vi "singleChannelGraphs_1.vi"(8 "Locations-IR 2":dbl[][](array[numeric])=[[0.0, 0.0, 0.0, 0.0, 0.0, 0.0, 0.0, 0.0, 0.0, 0.0, 0.0], [0.0, 0.0, 0.0, 0.0, 0.0, 0.0, 0.0, 0.0, 0.0, 0.0, 0.0], [0.0, 0.0, 0.0, 0.0, 0.0, 0.0, 0.0, 0.0, 0.0, 0.0, 0.0], [0.0, 0.0, 0.0, 0.0, 0.0, 0.0, 0.0, 0.0, 0.0, 0.0, 0.0], [1003.5977793333972, 1010.2987872733909, 1047.7043573372093, 1054.0581575907959, 1060.2441183129574, 1066.4237494286472, 1072.6076798246322, 1078.8502256474524, 1119.8606859005151, 1131.4795052552802, 1142.8109565689153], [0.0, 0.0, 0.0, 0.0, 0.0, 0.0, 0.0, 0.0, 0.0, 0.0, 0.0], [8947.909400008684, 0.0, 0.0, 0.0, 0.0, 0.0, 0.0, 0.0, 0.0, 0.0, 0.0], [0.0, 0.0, 0.0, 0.0, 0.0, 0.0, 0.0, 0.0, 0.0, 0.0, 0.0], [0.0, 0.0, 0.0, 0.0, 0.0, 0.0, 0.0, 0.0, 0.0, 0.0, 0.0], [0.0, 0.0, 0.0, 0.0, 0.0, 0.0, 0.0, 0.0, 0.0, 0.0, 0.0], [0.0, 0.0, 0.0, 0.0, 0.0, 0.0, 0.0, 0.0, 0.0, 0.0, 0.0], [0.0, 0.0, 0.0, 0.0, 0.0, 0.0, 0.0, 0.0, 0.0, 0.0, 0.0], [0.0, 0.0, 0.0, 0.0, 0.0, 0.0, 0.0, 0.0, 0.0, 0.0, 0.0], [0.0, 0.0, 0.0, 0.0, 0.0, 0.0, 0.0, 0.0, 0.0, 0.0, 0.0]], 9 "Locations-IR 1":dbl[][](array[numeric])=[[0.0, 0.0, 0.0, 0.0, 0.0, 0.0, 0.0, 0.0, 0.0, 0.0, 0.0, 0.0, 0.0, 0.0, 0.0, 0.0, 0.0, 0.0, 0.0, 0.0, 0.0, 0.0, 0.0, 0.0], [0.0, 0.0, 0.0, 0.0, 0.0, 0.0, 0.0, 0.0, 0.0, 0.0, 0.0, 0.0, 0.0, 0.0, 0.0, 0.0, 0.0, 0.0, 0.0, 0.0, 0.0, 0.0, 0.0, 0.0], [0.0, 0.0, 0.0, 0.0, 0.0, 0.0, 0.0, 0.0, 0.0, 0.0, 0.0, 0.0, 0.0, 0.0, 0.0, 0.0, 0.0, 0.0, 0.0, 0.0, 0.0, 0.0, 0.0, 0.0], [0.0, 0.0, 0.0, 0.0, 0.0, 0.0, 0.0, 0.0, 0.0, 0.0, 0.0, 0.0, 0.0, 0.0, 0.0, 0.0, 0.0, 0.0, 0.0, 0.0, 0.0, 0.0, 0.0, 0.0], [0.0, 0.0, 0.0, 0.0, 0.0, 0.0, 0.0, 0.0, 0.0, 0.0, 0.0, 0.0, 0.0, 0.0, 0.0, 0.0, 0.0, 0.0, 0.0, 0.0, 0.0, 0.0, 0.0, 0.0], [1949.3968989382124, 8950.779704911463, 0.0, 0.0, 0.0, 0.0, 0.0, 0.0, 0.0, 0.0, 0.0, 0.0, 0.0, 0.0, 0.0, 0.0, 0.0, 0.0, 0.0, 0.0, 0.0, 0.0, 0.0, 0.0], [1922.6824130689417, 1927.4536577782014, 8945.1544536163, 0.0, 0.0, 0.0, 0.0, 0.0, 0.0, 0.0, 0.0, 0.0, 0.0, 0.0, 0.0, 0.0, 0.0, 0.0, 0.0, 0.0, 0.0, 0.0, 0.0, 0.0], [8944.05693493819, 0.0, 0.0, 0.0, 0.0, 0.0, 0.0, 0.0, 0.0, 0.0, 0.0, 0.0, 0.0, 0.0, 0.0, 0.0, 0.0, 0.0, 0.0, 0.0, 0.0, 0.0, 0.0, 0.0], [1828.0609508803298, 1840.7040446097299, 1846.0822777647768, 1851.546050134507, 1859.188023533712, 1880.890963654859, 8946.459150564613, 0.0, 0.0, 0.0, 0.0, 0.0, 0.0, 0.0, 0.0, 0.0, 0.0, 0.0, 0.0, 0.0, 0.0, 0.0, 0.0, 0.0], [1003.8836135739322, 1034.6023970013964, 1053.8529427226035, 1059.3332515391548, 1066.1957876120568, 1101.2443464523667, 1107.1271826334205, 1113.3003458195556, 1124.7988705144635, 1158.4306678463795, 1163.8291284517709, 1174.9323436186403, 1222.5151135054907, 1227.7098546004795, 1278.1537733001408, 1789.4645001942506, 1803.3995277539998, 1813.0755151476708, 1815.1158947507906, 1827.5667796787511, 1840.7614524568564, 7629.760547014096, 8952.76455905497, 9371.69731664426], [1786.270481148661, 1790.662343187161, 1799.7774170223831, 0.0, 0.0, 0.0, 0.0, 0.0, 0.0, 0.0, 0.0, 0.0, 0.0, 0.0, 0.0, 0.0, 0.0, 0.0, 0.0, 0.0, 0.0, 0.0, 0.0, 0.0], [1758.269290749024, 1768.7972022285298, 1773.1698271444452, 1779.905620445401, 1785.2748566498417, 1797.4164166157257, 0.0, 0.0, 0.0, 0.0, 0.0, 0.0, 0.0, 0.0, 0.0, 0.0, 0.0, 0.0, 0.0, 0.0, 0.0, 0.0, 0.0, 0.0], [1731.9130549197157, 1741.9528957065543, 1746.8638380092243, 1756.4292982249558, 1769.4936601847248, 1775.4511666930466, 1785.5242437749614, 0.0, 0.0, 0.0, 0.0, 0.0, 0.0, 0.0, 0.0, 0.0, 0.0, 0.0, 0.0, 0.0, 0.0, 0.0, 0.0, 0.0], [1670.107666290024, 1721.118225421893, 1731.7339852624614, 1741.1929011419254, 1747.322588791405, 1755.3693388267866, 1763.3171095427958, 1768.6483249049165, 0.0, 0.0, 0.0, 0.0, 0.0, 0.0, 0.0, 0.0, 0.0, 0.0, 0.0, 0.0, 0.0, 0.0, 0.0, 0.0]], 10 "micro 1":dbl[][](array[numeric])=array14x10000[140000 elements], 11 "micro 2":dbl[][](array[numeric])=array14x10000[140000 elements]) -> ()   [LabVIEW 2014]
panel:
  in  "Numerisch":i32=30
  in  "Registerkarte":enum32{"micro 2", "micro 1"}(tab)=enum."micro 1"
  out "Gap_L11":dbl[][](graph)
  out "Gap_L10":dbl[][](graph)
  out "Gap_L9":dbl[][](graph)
  out "Gap_L8":dbl[][](graph)
  out "Gap_L7":dbl[][](graph)
  out "Gap_L6":dbl[][](graph)
  out "Gap_L5":dbl[][](graph)
  out "Gap_L4":dbl[][](graph)
  out "Gap_L3":dbl[][](graph)
  out "Gap_L1":dbl[][](graph)
  out "Gap_L2":dbl[][](graph)
  out "Gap_L12":dbl[][](graph)
  out "Gap_L13":dbl[][](graph)
  out "Gap_L14":dbl[][](graph)
  out "Gap_R11":dbl[][](graph)
  out "Gap_R10":dbl[][](graph)
  out "Gap_R9":dbl[][](graph)
  out "Gap_R8":dbl[][](graph)
  out "Gap_R6":dbl[][](graph)
  out "Gap_R5":dbl[][](graph)
  out "Gap_R4":dbl[][](graph)
  out "Speaker R3":dbl[][](graph)
  out "Gap_R7":dbl[][](graph)
  out "Speaker R1":dbl[](graph)
  out "Speaker R2":dbl[](graph)
  out "Speaker R14":dbl[](graph)
  out "Gap_R11 2":dbl[][](graph)
  out "Gap_R13":dbl[][](graph)
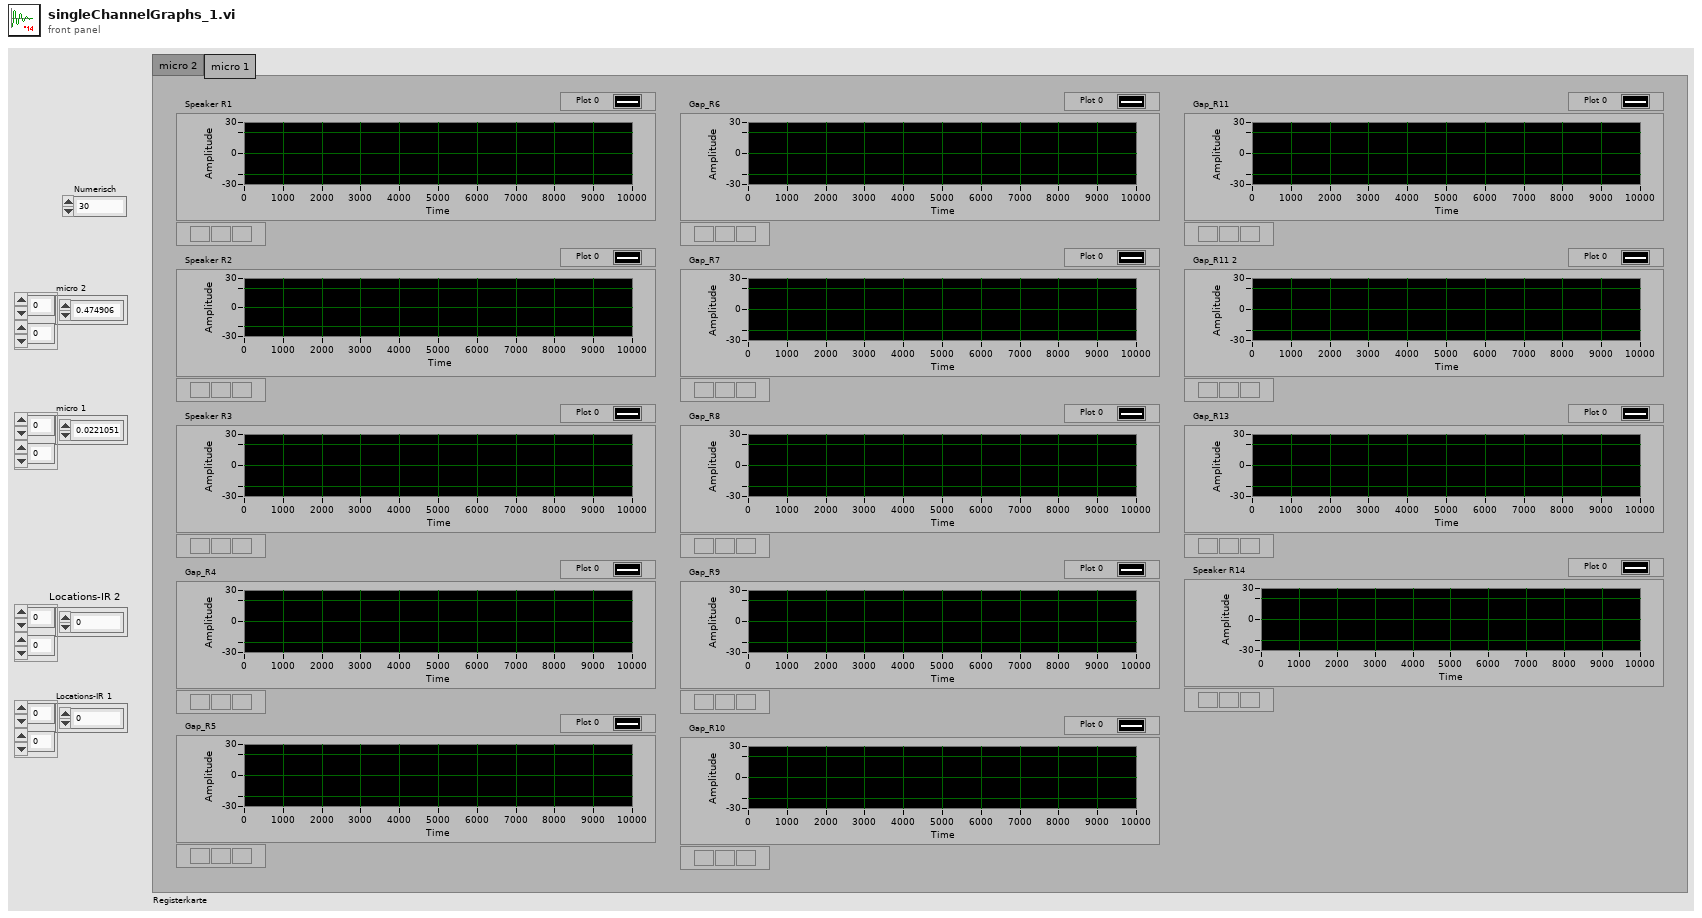
[diagram p1: front panel]
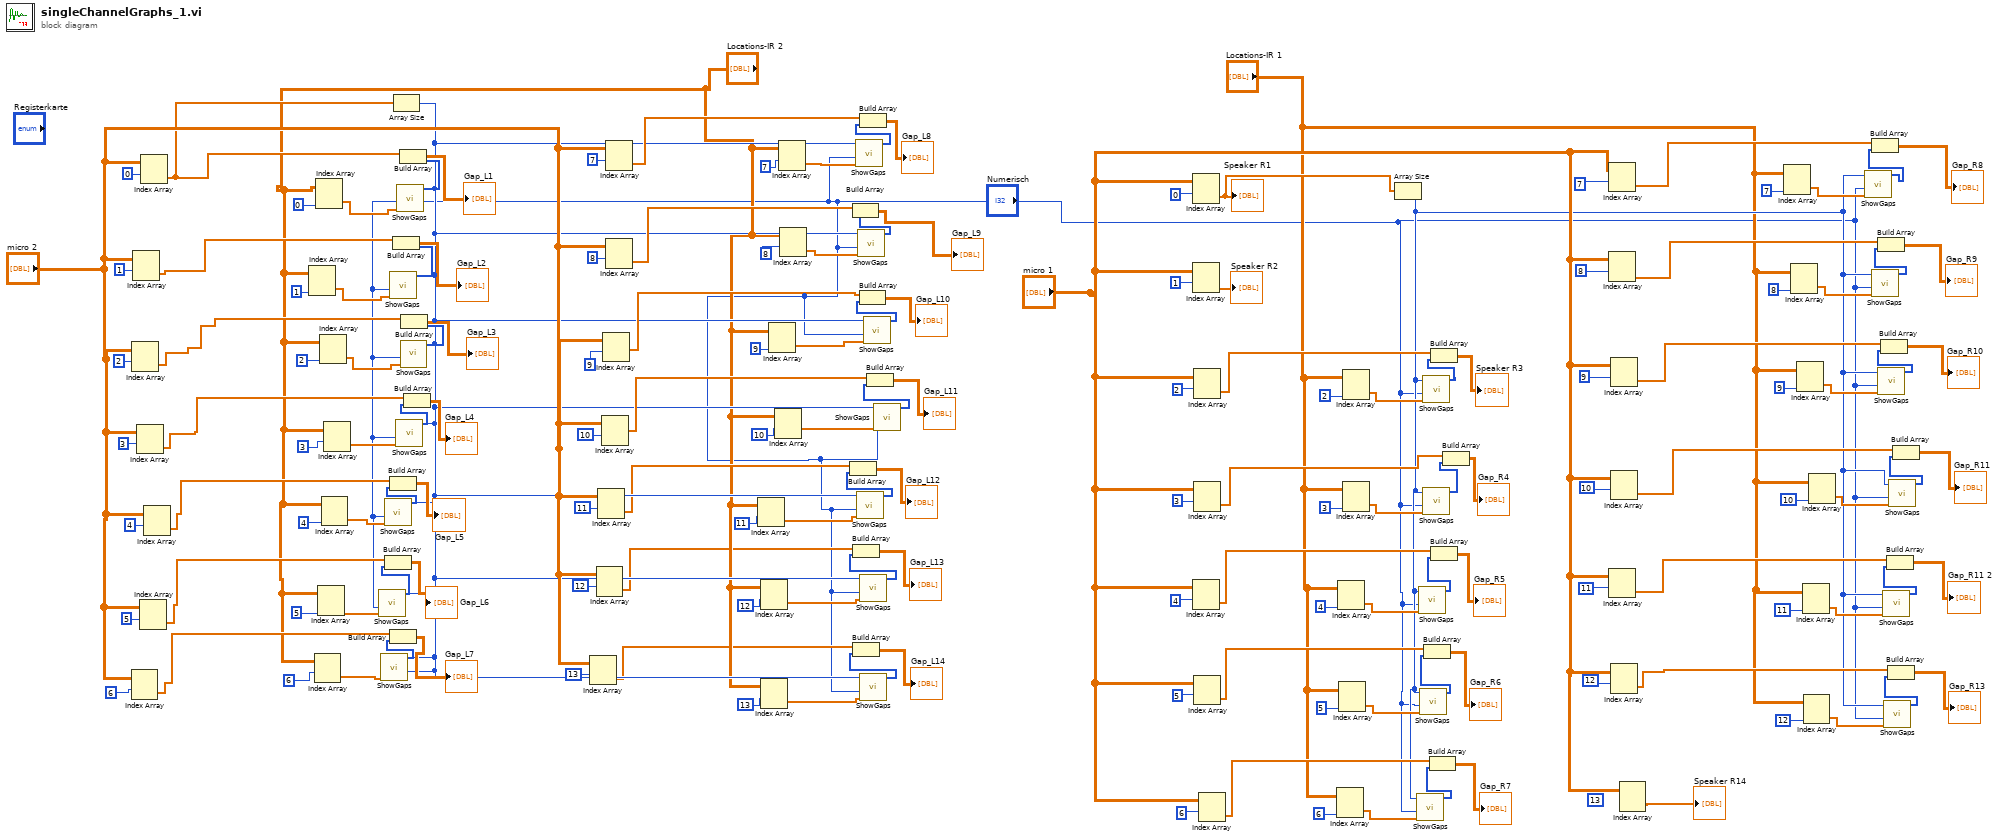
[diagram p0: block diagram]
diagram:
  (unwired) 13
  n1 = Index Array(array="micro 2", index (row)=6) -> (element=w82:dbl[])  [unwired: 1 in]
  n2 = Index Array(array="micro 2", index (row)=2) -> (element=w94:dbl[])  [unwired: 1 in]
  n3 = Index Array(array="micro 2", index (row)=1) -> (element=w20:dbl[])  [unwired: 1 in]
  n4 = Index Array(array="micro 2", index (row)=3) -> (element=w91:dbl[])  [unwired: 1 in]
  n5 = Index Array(array="micro 2", index (row)=5) -> (element=w85:dbl[])  [unwired: 1 in]
  n6 = Index Array(array="micro 2", index (row)=0) -> (element=w21:dbl[])  [unwired: 1 in]
  n7 = Index Array(array="micro 2", index (row)=4) -> (element=w88:dbl[])  [unwired: 1 in]
  n8 = Index Array(array="Locations-IR 2", index (row)=1 ("Index (Spalte)")) -> (element=w24:dbl[])  [unwired: 1 in]
  n9 = Index Array(array="Locations-IR 2", index (row)=6 ("Index (Spalte)")) -> (element=w118:dbl[])  [unwired: 1 in]
  n10 = Index Array(array="Locations-IR 2", index (row)=0 ("Index (Spalte)")) -> (element=w27:dbl[])  [unwired: 1 in]
  n11 = Index Array(array="Locations-IR 2", index (row)=5 ("Index (Spalte)")) -> (element=w119:dbl[])  [unwired: 1 in]
  n12 = Index Array(array="Locations-IR 2", index (row)=2 ("Index (Spalte)")) -> (element=w122:dbl[])  [unwired: 1 in]
  n13 = Index Array(array="Locations-IR 2", index (row)=4 ("Index (Spalte)")) -> (element=w120:dbl[])  [unwired: 1 in]
  n14 = Index Array(array="Locations-IR 2", index (row)=3 ("Index (Spalte)")) -> (element=w121:dbl[])  [unwired: 1 in]
  n15 = Array Size(array=w21) -> (size(s)=w9:i32)
  n16 = call "ShowGaps.vi"("peaklocations"=w119, "Numerisch"="Numerisch", "length of IR"=w9) -> ("ShowGap"=w84:i32[])  [unwired: 8 in]
  n17 = call "ShowGaps.vi"("peaklocations"=w118, "Numerisch"=w9, "length of IR"=w9) -> ("ShowGap"=w81:i32[])  [unwired: 8 in]
  n18 = call "ShowGaps.vi"("peaklocations"=w120, "Numerisch"="Numerisch", "length of IR"=w9) -> ("ShowGap"=w87:i32[])  [unwired: 8 in]
  n19 = Build Array(w85, w84) -> (→"Gap_L6":dbl[][])
  n20 = call "ShowGaps.vi"("peaklocations"=w24, "Numerisch"="Numerisch", "length of IR"=w9) -> ("ShowGap"=w23:i32[])  [unwired: 8 in]
  n21 = Build Array(w88, w87) -> (→"Gap_L5":dbl[][])
  n22 = Build Array(w82, w81) -> (→"Gap_L7":dbl[][])
  n23 = Build Array(w20, w23) -> (→"Gap_L2":dbl[][])
  n24 = call "ShowGaps.vi"("peaklocations"=w121, "Numerisch"="Numerisch", "length of IR"=w9) -> ("ShowGap"=w90:i32[])  [unwired: 8 in]
  n25 = call "ShowGaps.vi"("peaklocations"=w27, "length of IR"=w9) -> ("ShowGap"=w26:i32[])  [unwired: 9 in]
  n26 = Build Array(w21, w26) -> (→"Gap_L1":dbl[][])
  n27 = call "ShowGaps.vi"("peaklocations"=w122, "Numerisch"="Numerisch", "length of IR"=w9) -> ("ShowGap"=w93:i32[])  [unwired: 8 in]
  n28 = Build Array(w94, w93) -> (→"Gap_L3":dbl[][])
  n29 = Build Array(w91, w90) -> (→"Gap_L4":dbl[][])
  n30 = Index Array(array="micro 2", index (row)=13) -> (element=w6:dbl[])  [unwired: 1 in]
  n31 = Index Array(array="micro 2", index (row)=12) -> (element=w5:dbl[])  [unwired: 1 in]
  n32 = Index Array(array="micro 2", index (row)=11) -> (element=w8:dbl[])  [unwired: 1 in]
  n33 = Index Array(array="micro 2", index (row)=10) -> (element=w70:dbl[])  [unwired: 1 in]
  n34 = Index Array(array="micro 2", index (row)=9) -> (element=w73:dbl[])  [unwired: 1 in]
  n35 = Index Array(array="micro 2", index (row)=7) -> (element=w79:dbl[])  [unwired: 1 in]
  n36 = Index Array(array="micro 2", index (row)=8) -> (element=w76:dbl[])  [unwired: 1 in]
  n37 = Index Array(array="Locations-IR 2", index (row)=11 ("Index (Spalte)")) -> (element=w3:dbl[])  [unwired: 1 in]
  n38 = Index Array(array="Locations-IR 2", index (row)=12 ("Index (Spalte)")) -> (element=w4:dbl[])  [unwired: 1 in]
  n39 = Index Array(array="Locations-IR 2", index (row)=13 ("Index (Spalte)")) -> (element=w2:dbl[])  [unwired: 1 in]
  n40 = Index Array(array="Locations-IR 2", index (row)=9 ("Index (Spalte)")) -> (element=w116:dbl[])  [unwired: 1 in]
  n41 = Index Array(array="Locations-IR 2", index (row)=10 ("Index (Spalte)")) -> (element=w117:dbl[])  [unwired: 1 in]
  n42 = Index Array(array="Locations-IR 2", index (row)=7 ("Index (Spalte)")) -> (element=w114:dbl[])  [unwired: 1 in]
  n43 = Index Array(array="Locations-IR 2", index (row)=8 ("Index (Spalte)")) -> (element=w115:dbl[])  [unwired: 1 in]
  n44 = call "ShowGaps.vi"("peaklocations"=w114, "Numerisch"="Numerisch", "length of IR"=w9) -> ("ShowGap"=w78:i32[])  [unwired: 8 in]
  n45 = call "ShowGaps.vi"("peaklocations"=w3, "Numerisch"="Numerisch", "length of IR"=w9) -> ("ShowGap"=w17:i32[])  [unwired: 8 in]
  n46 = Build Array(w8, w17) -> (→"Gap_L12":dbl[][])
  n47 = call "ShowGaps.vi"("peaklocations"=w115, "Numerisch"="Numerisch", "length of IR"=w9) -> ("ShowGap"=w75:i32[])  [unwired: 8 in]
  n48 = Build Array(w76, w75) -> (→"Gap_L9":dbl[][])
  n49 = Build Array(w79, w78) -> (→"Gap_L8":dbl[][])
  n50 = call "ShowGaps.vi"("peaklocations"=w4, "Numerisch"="Numerisch", "length of IR"=w9) -> ("ShowGap"=w14:i32[])  [unwired: 8 in]
  n51 = Build Array(w5, w14) -> (→"Gap_L13":dbl[][])
  n52 = call "ShowGaps.vi"("peaklocations"=w2, "Numerisch"="Numerisch", "length of IR"=w9) -> ("ShowGap"=w11:i32[])  [unwired: 8 in]
  n53 = Build Array(w6, w11) -> (→"Gap_L14":dbl[][])
  n54 = call "ShowGaps.vi"("peaklocations"=w116, "Numerisch"="Numerisch", "length of IR"=w9) -> ("ShowGap"=w72:i32[])  [unwired: 8 in]
  n55 = Build Array(w73, w72) -> (→"Gap_L10":dbl[][])
  n56 = call "ShowGaps.vi"("peaklocations"=w117, "Numerisch"="Numerisch", "length of IR"=w9) -> ("ShowGap"=w69:i32[])  [unwired: 8 in]
  n57 = Build Array(w70, w69) -> (→"Gap_L11":dbl[][])
  n58 = Index Array(array="micro 1", index (row)=0) -> (element=w95:dbl[])  [unwired: 1 in]
  "Speaker R1" <- w95
  n59 = Index Array(array="micro 1", index (row)=1) -> (element=→"Speaker R2":dbl[])  [unwired: 1 in]
  n60 = Index Array(array="micro 1", index (row)=4) -> (element=w61:dbl[])  [unwired: 1 in]
  n61 = Index Array(array="micro 1", index (row)=2) -> (element=w67:dbl[])  [unwired: 1 in]
  n62 = Index Array(array="micro 1", index (row)=3) -> (element=w64:dbl[])  [unwired: 1 in]
  n63 = Index Array(array="micro 1", index (row)=5) -> (element=w58:dbl[])  [unwired: 1 in]
  n64 = Index Array(array="micro 1", index (row)=6) -> (element=w55:dbl[])  [unwired: 1 in]
  n65 = Index Array(array="Locations-IR 1", index (row)=6 ("Index (Spalte)")) -> (element=w104:dbl[])  [unwired: 1 in]
  n66 = Index Array(array="Locations-IR 1", index (row)=4 ("Index (Spalte)")) -> (element=w108:dbl[])  [unwired: 1 in]
  n67 = Index Array(array="Locations-IR 1", index (row)=5 ("Index (Spalte)")) -> (element=w106:dbl[])  [unwired: 1 in]
  n68 = Index Array(array="Locations-IR 1", index (row)=2 ("Index (Spalte)")) -> (element=w112:dbl[])  [unwired: 1 in]
  n69 = Index Array(array="Locations-IR 1", index (row)=3 ("Index (Spalte)")) -> (element=w110:dbl[])  [unwired: 1 in]
  n70 = Array Size(array=w95) -> (size(s)=w30:i32)
  n71 = call "ShowGaps.vi"("peaklocations"=w104, "Numerisch"="Numerisch", "length of IR"=w30) -> ("ShowGap"=w54:i32[])  [unwired: 8 in]
  n72 = call "ShowGaps.vi"("peaklocations"=w108, "Numerisch"="Numerisch", "length of IR"=w30) -> ("ShowGap"=w60:i32[])  [unwired: 8 in]
  n73 = call "ShowGaps.vi"("peaklocations"=w106, "Numerisch"="Numerisch", "length of IR"=w30) -> ("ShowGap"=w57:i32[])  [unwired: 8 in]
  n74 = call "ShowGaps.vi"("peaklocations"=w112, "Numerisch"="Numerisch", "length of IR"=w30) -> ("ShowGap"=w66:i32[])  [unwired: 8 in]
  n75 = call "ShowGaps.vi"("peaklocations"=w110, "Numerisch"="Numerisch", "length of IR"=w30) -> ("ShowGap"=w63:i32[])  [unwired: 8 in]
  n76 = Build Array(w58, w57) -> (→"Gap_R6":dbl[][])
  n77 = Build Array(w55, w54) -> (→"Gap_R7":dbl[][])
  n78 = Build Array(w67, w66) -> (→"Speaker R3":dbl[][])
  n79 = Build Array(w61, w60) -> (→"Gap_R5":dbl[][])
  n80 = Build Array(w64, w63) -> (→"Gap_R4":dbl[][])
  n81 = Index Array(array="micro 1", index (row)=7) -> (element=w52:dbl[])  [unwired: 1 in]
  n82 = Index Array(array="micro 1", index (row)=8) -> (element=w49:dbl[])  [unwired: 1 in]
  n83 = Index Array(array="micro 1", index (row)=11) -> (element=w36:dbl[])  [unwired: 1 in]
  n84 = Index Array(array="micro 1", index (row)=9) -> (element=w46:dbl[])  [unwired: 1 in]
  n85 = Index Array(array="micro 1", index (row)=10) -> (element=w43:dbl[])  [unwired: 1 in]
  n86 = Index Array(array="micro 1", index (row)=12) -> (element=w31:dbl[])  [unwired: 1 in]
  n87 = Index Array(array="micro 1") -> (element=→"Speaker R14":dbl[])  [unwired: 2 in]
  n88 = Index Array(array="Locations-IR 1", index (row)=7 ("Index (Spalte)")) -> (element=w102:dbl[])  [unwired: 1 in]
  n89 = Index Array(array="Locations-IR 1", index (row)=8 ("Index (Spalte)")) -> (element=w100:dbl[])  [unwired: 1 in]
  n90 = Index Array(array="Locations-IR 1", index (row)=9 ("Index (Spalte)")) -> (element=w98:dbl[])  [unwired: 1 in]
  n91 = Index Array(array="Locations-IR 1", index (row)=11 ("Index (Spalte)")) -> (element=w39:dbl[])  [unwired: 1 in]
  n92 = Index Array(array="Locations-IR 1", index (row)=12 ("Index (Spalte)")) -> (element=w34:dbl[])  [unwired: 1 in]
  n93 = Index Array(array="Locations-IR 1", index (row)=10 ("Index (Spalte)")) -> (element=w96:dbl[])  [unwired: 1 in]
  n94 = call "ShowGaps.vi"("peaklocations"=w102, "Numerisch"="Numerisch", "length of IR"=w30) -> ("ShowGap"=w51:i32[])  [unwired: 8 in]
  n95 = Build Array(w52, w51) -> (→"Gap_R8":dbl[][])
  n96 = call "ShowGaps.vi"("peaklocations"=w100, "Numerisch"="Numerisch", "length of IR"=w30) -> ("ShowGap"=w48:i32[])  [unwired: 8 in]
  n97 = Build Array(w49, w48) -> (→"Gap_R9":dbl[][])
  n98 = call "ShowGaps.vi"("peaklocations"=w98, "Numerisch"="Numerisch", "length of IR"=w30) -> ("ShowGap"=w45:i32[])  [unwired: 8 in]
  n99 = Build Array(w46, w45) -> (→"Gap_R10":dbl[][])
  n100 = call "ShowGaps.vi"("peaklocations"=w39, "Numerisch"="Numerisch", "length of IR"=w30) -> ("ShowGap"=w38:i32[])  [unwired: 8 in]
  n101 = call "ShowGaps.vi"("peaklocations"=w34, "Numerisch"="Numerisch", "length of IR"=w30) -> ("ShowGap"=w33:i32[])  [unwired: 8 in]
  n102 = Build Array(w36, w38) -> (→"Gap_R11 2":dbl[][])
  n103 = Build Array(w31, w33) -> (→"Gap_R13":dbl[][])
  n104 = call "ShowGaps.vi"("peaklocations"=w96, "Numerisch"="Numerisch", "length of IR"=w30) -> ("ShowGap"=w42:i32[])  [unwired: 8 in]
  n105 = Build Array(w43, w42) -> (→"Gap_R11":dbl[][])
